vi "HFRR ADV v039.vi"() -> ()   [LabVIEW 2025] (continued)
    n1697 = local read "Calibration Tare Value"() -> (w2060:dbl)
    n1698 = local read "Calibration Tare"() -> (w2058:bool)
    n1699 = Subtract(x=w2056, y=w2060) -> (x-y=→"LVDT STROKE  Calibration":dbl)
    n1700 = case shown="True" w2058 {
      selector: w2058 -> [_ w2066]
      tunnel: w2056 -> [_ w2067]
      frame False {
      }
      frame True {
        n1701 = Not(x=w2066) -> (.not. x?=w2065:bool)
        n1702 = local write "Calibration Tare"(w2065) -> ()
        "Calibration Tare Value" <- w2067
      }
    }
    n1703 = local read "Quit"() -> (w2064:bool)
  }
  n1704 = while {
    stop <- w2090 stop-if-true
    n1705 = local read "Due read"() -> (w2088:string)
    n1706 = call <vilib>:"High Resolution Polling Wait.vi"("seconds to wait"=0.02) -> ()  [unwired: 10 in, 1 out]
    n1707 = local read "Frictioin Force Raw"() -> (w2070:dbl)
    n1708 = Spreadsheet String To Array(delimiter (Tab)=";", format string="", spreadsheet string=w2088, array type (2D Dbl)=string[] []) -> (array=w2085:string[])
    n1709 = Fract/Exp String To Number(string=w2085) -> (number=w2084:dbl[])  [unwired: 3 in, 1 out]
    n1710 = call <vilib>:"Median Filter PtByPt.vi"("rank"=2, "x"=w2070) -> ("Filtered x"=→"Friction":dbl)  [unwired: 2 in, 1 out]
    n1711 = Index Array(array=w2084) -> (element #1=→"Sample Temperature":dbl, element #2=→"Target Sample Temperature":dbl, element #3=→"Current Duty Cycle":dbl, element #4=→"Ambient Temperature":dbl, element #5=→"Dac Status":dbl, element #6=→"Vpp":dbl, element #7=→"Active Error Code":dbl, element #8=→"Kp":dbl, element #9=→"Ki":dbl, element #10=→"Kd":dbl, element #11=→"SampleRaw":dbl, element #12=→"AmbRaw":dbl)  [unwired: 12 in]
    n1712 = local read "Quit"() -> (w2090:bool)
  }
  n1713 = while {
    shift-right: [w2104] -> w41
    shift-left: _ -> [w2096]
    shift-right: [w2091] -> w40
    shift-left: errorcluster {"status"=FALSE, "code"=0, "source"="Init"} ("error out") -> [w2098]
    tunnel: [w2093] -> w44
    tunnel: [w2103] -> _
    i -> [w2103]
    stop <- w2093 stop-if-true
    n1714 = local read "Com Port 2"() -> (w2097:refnum<visa-resource-name>)
    n1715 = local read "Port 2a"() -> (w2099:bool)
    n1716 = Unbundle(w2098) -> ("status"=→"Port 4":bool)  [unwired: 2 out]
    n1717 = call <vilib>:"High Resolution Polling Wait.vi"("seconds to wait"=0.02) -> ()  [unwired: 10 in, 1 out]
    n1718 = local read "Port 4"() -> (w2100:bool)
    n1719 = Not Equal?(x=w2097, y=w2096) -> (x != y?=w2095:bool)
    n1720 = Or(x=w2100, y=w2099) -> (x .or. y?=w2102:bool)
    n1721 = case shown="False" w2102 {
      frame False {
        w2107 = TRUE ("Visible")
        n1722 = property on="Port 2a" class="Bool (strict)"("Visible"=w2107) -> ()  [unwired: 2 in, 2 out]
        n1723 = property on="Port 4" class="Bool (strict)"("Visible"=w2107) -> ()  [unwired: 2 in, 2 out]
      }
      frame True {
        w2108 = TRUE ("Visible")
        n1724 = property on="Port 2a" class="Bool (strict)"("Visible"=w2108) -> ()  [unwired: 2 in, 2 out]
        n1725 = property on="Port 4" class="Bool (strict)"("Visible"=w2108) -> ()  [unwired: 2 in, 2 out]
      }
    }
    n1726 = case shown="True" w2095 {
      tunnel: [w2105 errorcluster {"status"=TRUE, "code"=0, "source"="Init"} ("error out")] -> w2094
      tunnel: w2098 -> [w2105 _]
      frame False {
      }
      frame True {
      }
    }
    n1727 = case shown="No Error" w2094 {
      selector: w2094 -> [w2121 w2152]
      tunnel: [w2114 w2157] -> w2104
      tunnel: [w2122 w2150] -> w2091
      tunnel: w2096 -> [w2123 w2155]
      frame No Error {
        n1728 = property class="Instr" props=["Serial Settings:Number of Bytes at Serial Port"](reference=w2123, error in=w2121) -> (reference out=w2115:refnum<visa-resource-name>, error out=w2120:errorcluster)  [unwired: 1 out]
        n1729 = while {
          tunnel: [w2131] -> w2116
          tunnel: [w2130] -> w2117
          tunnel: w2120 -> [w2129]
          tunnel: w2115 -> [w2128]
          tunnel: [w2127] -> _
          i -> [w2127]
          stop <- TRUE stop-if-true
          n1730 = property class="Instr" props=["Serial Settings:Number of Bytes at Serial Port"](reference=w2128, error in=w2129) -> (reference out=w2133:refnum<visa-resource-name>, error out=w2132:errorcluster)  [unwired: 1 out]
          n1731 = VISA Read(VISA resource name=w2133, byte count=u32 1000, error in (no error)=w2132) -> (VISA resource name out=w2130:refnum<visa-resource-name>, read buffer=→"Due read":string, error out=w2131:errorcluster)  [unwired: 1 out]
        }
        n1732 = local read "Due Write"() -> (w2113:string)
        n1733 = call <vilib>:"Trim Whitespace.vi"("string"=w2113) -> ("trimmed string"=w2112:string)  [unwired: 1 in]
        n1734 = Not Equal?(x=w2112, y="") -> (x != y?=w2118:bool)
        n1735 = VISA Flush I/O Buffer(VISA resource name=w2117) -> (VISA resource name out=w2110:refnum<visa-resource-name>, error out=→"error out 10":errorcluster)  [unwired: 2 in]
        n1736 = case shown="True" w2118 {
          tunnel: w2110 -> [w2135 w2140]
          tunnel: [w2135 w2144] -> w2114
          tunnel: w2116 -> [w2134 w2139]
          tunnel: [w2134 w2142] -> w2122
          tunnel: w2112 -> [_ w2138]
          tunnel: [_ w2141] -> _
          frame False {
            # "DATA  WRITE LOOP"
          }
          frame True {
            n1737 = Concatenate Strings(w2138, "\r\n") -> (w2137:string)
            n1738 = VISA Write(VISA resource name=w2140, write buffer=w2137, error in (no error)=w2139) -> (VISA resource name out=w2144:refnum<visa-resource-name>, return count=w2141:u32, error out=w2143:errorcluster)
            n1739 = flat-sequence {
              tunnel: w2143 -> [w2146]
              tunnel: [w2146] -> w2142
              frame #0 {
                n1740 = local write "Due Write"("" ("Command")) -> ()
                n1741 = Wait (ms)(milliseconds to wait=u32 5) -> ()  [unwired: 1 out]
              }
            }
          }
        }
        "Port 2a" <- TRUE ("Port 2a")
      }
      frame Error {
        w2163 = u16 0 items=["None", "XON/XOFF", "RTS/CTS", "XON/XOFF & RTS/CTS", "DTR/DSR", "XON/XOFF & DTR/DSR"] ("flow control (0:none)  2")
        w2161 = u16 10 items=["1.0"=10, "1.5"=15, "2.0"=20] ("stop bits 2")
        w2159 = u16 0 items=["None", "Odd", "Even", "Mark", "Space"] ("parity 2")
        w2160 = u32 10000  # timeout (10sec)
        n1742 = VISA Clear(VISA resource name=w2155, error in (no error)=w2152) -> (VISA resource name out=w2154:refnum<visa-resource-name>, error out=w2153:errorcluster)
        n1743 = VISA Close(VISA resource name=w2154, error in (no error)=w2153) -> (error out=w2156:errorcluster)
        n1744 = call <vilib>:"Clear Errors.vi"("error in (no error)"=w2156) -> ()  [unwired: 5 in, 2 out]
        n1745 = local write "Port 2a"(FALSE ("Port 2a")) -> ()
        n1746 = local read "Com Port 2"() -> (w2149:refnum<visa-resource-name>)
        "visa due" <- w2149
        n1747 = call-poly "VISA Configure Serial Port"("VISA resource name"=w2149, "timeout (10sec)"=w2160, "baud rate (9600)"=u32 250000 ("baud rate  2"), "data bits (8)"=u16 8 ("data bits  2"), "parity (0:none)"=w2159, "stop bits (10: 1 bit)"=w2161, "flow control (0:none)"=w2163) -> ("VISA resource name out"=w2164:refnum<visa-resource-name>, "error out"=w2165:errorcluster)  [unwired: 7 in]
        n1748 = flat-sequence {
          tunnel: w2164 -> [w2167]
          tunnel: w2165 -> [w2166]
          tunnel: [w2167] -> w2157
          tunnel: [w2166] -> w2150
          frame #0 {
            n1749 = Wait (ms)(milliseconds to wait=u32 50) -> ()  [unwired: 1 out]
          }
        }
        "Residual Due" <- ""
      }
    }
    "error out 9" <- w2091
    n1750 = local read "Quit"() -> (w2093:bool)
    "Error Due" <- w2098
  }
  n1751 = local write "FRICVALZ"(0.0 ("FRICVALZ")) -> ()
  n1752 = property on="RUN" class="Bool (strict)"("Visible"=TRUE) -> ()  [unwired: 2 in, 2 out]
  n1753 = while {
    tunnel: [w2182] -> _
    tunnel: [w2169] -> w54
    i -> [w2182]
    stop <- w2169 stop-if-true
    n1754 = local read "conststatus"() -> (w2173:dbl)
    n1755 = local read "Main Tab"() -> (w2171:T2)
    n1756 = local read "EDIT"() -> (w2188:bool)
    n1757 = local read "Rate"() -> (w2187:dbl)
    n1758 = case shown="True" w2188 {
      tunnel: [FALSE TRUE] -> _
      frame False {
      }
      frame True {
      }
    }
    n1759 = Equal?(x=w2171, y=T29."About" ("Main Tab")) -> (x = y?=w2180:bool)
    n1760 = Equal?(x=w2173, y=0.0) -> (x = y?=w2174:bool)
    n1761 = Divide(x=1.0, y=w2187) -> (x/y=w2183:dbl)
    "Time 2" <- w2183
    n1762 = case shown="True" w2174 {
      frame False {
      }
      frame True {
        # "C:\\WinDucom\\calibrate WO 2391.dcf"
        n1763 = local write "Lan flag"(22) -> ()
        n1764 = local write "conststatus"(10.0 ("rpm value : 2")) -> ()
        n1765 = String To Path(string="C:\\LAB-IQ\\calibrate WO 2465.dcf") -> (path=w2194:path)
        n1766 = Open/Create/Replace File "Open File"(file path (use dialog)=w2194) -> (refnum out=w2192:refnum<file>)  [unwired: 5 in, 2 out]
        n1767 = for {
          N: 23 -> [_]
          tunnel: w2192 -> [w2203]
          i -> [w2197]
          (unwired) TRUE ("line mode (F)")
          n1768 = Read from Text File "Read File"(file (use dialog)=w2203) -> (text=w2202:string)  [unwired: 3 in, 3 out]
          n1769 = Match Pattern(string=w2202, regular expression="]") -> (after substring=w2200:string)  [unwired: 1 in, 3 out]
          n1770 = String Subset(string=w2202, offset (0)=5, length (rest)=10 ("length (rest)")) -> (substring=w2195:string)
          n1771 = Fract/Exp String To Number(string=w2195) -> (number=w2196:dbl)  [unwired: 3 in, 1 out]
          n1772 = Match Pattern(string=w2200, regular expression="-") -> (before substring=w2198:string)  [unwired: 1 in, 3 out]
          n1773 = case shown="10" w2197 {
            tunnel: w2196 -> [_ _ _ _ _ _ _ _ _ _ w2210 _ _ _ _ _ _ _ _ _ _ _ _ _]
            tunnel: w2198 -> [_ _ _ _ w2206 w2207 w2208 _ _ _ _ _ _ _ _ _ _ _ _ _ w2211 w2212 w2213 _]
            frame 0 {
            }
            frame 1 {
            }
            frame 2 {
            }
            frame 3 {
            }
            frame 4 {
              n1774 = local write "Com Port 1"(w2206) -> ()
            }
            frame 5 {
              n1775 = local write "Com Port 2"(w2207) -> ()
              n1776 = local write "visa due"(w2207) -> ()
            }
            frame 6 {
              n1777 = String To Path(string=w2208) -> (path=w2209:path)
              n1778 = local write "File Path"(w2209) -> ()
              "String" <- w2208
            }
            frame 7 {
            }
            frame 8 {
            }
            frame 9 {
            }
            frame 10 {
              n1779 = local write "Language Selection"(w2210) -> ()
            }
            frame 11 {
            }
            frame 12 {
            }
            frame 13 {
            }
            frame 14 {
            }
            frame 15 {
            }
            frame 16 {
            }
            frame 17 {
            }
            frame 18 {
            }
            frame 21 {
            }
            frame 22 {
              n1780 = local write "Com Port 3"(w2211) -> ()
            }
            frame 20 {
              n1781 = local write "Camera Port :"(w2212) -> ()
            }
            frame 19 {
              n1782 = local write "C3 :"(w2213) -> ()
            }
            frame 23, Default {
            }
          }
        }
      }
    }
    n1783 = Select(t=u32 2500 ("milliseconds to wait"), s=w2180, f=u32 500 ("milliseconds to wait")) -> (s? t:f=w2178:u32)
    n1784 = Multiply(x=w2183, y=w2178) -> (x*y=w2185:dbl)
    n1785 = call "Elapsed Time2"("Time Target (s)"=w2185, "Auto Reset"=TRUE) -> ("Time has Elapsed"=w2175:bool)  [unwired: 10 in, 7 out]
    n1786 = case shown="True" w2175 {
      frame False {
      }
      frame True {
        n1787 = stacked-sequence {
          frame #0 {
            # "DATA PROCESSING"
            # "115 mV/N"
            n1788 = local read "Sample Temperature"() -> (w2216:dbl)
            n1789 = local read "RH Numeric:"() -> (→"Humidity ( %RH )":dbl)
            n1790 = local read "FRICVALZ"() -> (w2233:dbl)
            n1791 = local read "Friction"() -> (w2219:dbl)
            n1792 = call <vilib>:"Mean PtByPt.vi"("x"=w2216, "sample length"=100) -> ("mean"=w2215:dbl)  [unwired: 2 in, 1 out]
            "TEMP 2" <- w2215
            "TEMP 3" <- w2215
            n1793 = Subtract(x=w2219, y=w2233) -> (x-y=w2228:dbl)
            "FF 2" <- w2228
            "FF 4" <- w2228
            n1794 = local read "Ambient Temperature"() -> (→"AIR TEMP":dbl)
            n1795 = local read "TEMP"() -> (w2232:dbl)
            n1796 = local write "FF 3"(w2228) -> ()
            n1797 = Compound Arithmetic op=OR("FRICVALZ 4", "FRICVALZ 3", "FRICVALZ 2") -> (w2224:bool)
            n1798 = case shown="True" w2224 {
              tunnel: w2219 -> [_ w2239]
              frame False {
              }
              frame True {
                w2238 = FALSE ("FRICVALZ")
                n1799 = local write "FRICVALZ 3"(w2238) -> ()
                n1800 = local write "FRICVALZ 2"(w2238) -> ()
                n1801 = local write "FRICVALZ 4"(w2238) -> ()
                "FRICVALZ" <- w2239
              }
            }
            n1802 = Not A Number/Path/Refnum?(number/path/refnum=w2232) -> (NaN/Path/Refnum?=w2231:bool)
            n1803 = Not A Number/Path/Refnum?(number/path/refnum=w2228) -> (NaN/Path/Refnum?=w2230:bool)
            n1804 = Divide(x=w2228, y=1.96) -> (x/y=w2225:dbl)
            n1805 = Compound Arithmetic op=OR(w2231, w2230) -> (w2229:bool)
            n1806 = Not A Number/Path/Refnum?(number/path/refnum=w2225) -> (NaN/Path/Refnum?=w2226:bool)
            n1807 = case shown="True" w2229 {
              frame False {
              }
              frame True {
                n1808 = local write "TEMP"(0.0 ("TEMP")) -> ()
                n1809 = local write "FF 2"(0.0 ("FF 2")) -> ()
                n1810 = local write "reinit"(TRUE ("reinit")) -> ()
              }
            }
            n1811 = local write "TEMP"(w2215) -> ()
            n1812 = Select(t=0.0, s=w2226, f=w2225) -> (s? t:f=w2218:dbl)
            "COF 2" <- w2218
            n1813 = local write "COF 3"(w2218) -> ()
          }
        }
      }
    }
    n1814 = Wait (ms)(milliseconds to wait=u32 50) -> ()  [unwired: 1 out]
    n1815 = local read "Quit"() -> (w2169:bool)
    "Rate" <- 2500.0 ("No of Samples")
  }
  n1816 = while {
    tunnel: [w2259] -> _
    tunnel: [w2242] -> w56
    tunnel: w1 -> [_]
    i -> [w2259]
    stop <- w2242 stop-if-true
    # "C:\\LAB-IQ-NXT\\Scar View.exe"
    n1817 = local read "OK Button 16"() -> (w2249:bool)
    n1818 = local read "Main Tab"() -> (w2243:T2)
    n1819 = local read "service 3"() -> (w2244:bool)
    n1820 = local read "OPEN 6"() -> (w2246:bool)
    n1821 = local read "EDIT 2"() -> (w2248:bool)
    n1822 = flat-sequence {
      frame #0 {
        n1823 = stacked-sequence {
          frame #0 {
            n1824 = local read "EDIT"() -> (w2737:bool)
            n1825 = case shown="False" w2737 {
              tunnel: [u8 2 ("Disabled") u8 0 ("Disabled")] -> _
              frame False {
                w2739 = FALSE
                n1826 = local write "Password"("") -> ()
                n1827 = local write "x = y?"(w2739) -> ()
                n1828 = property on="Password" class="Str"("Visible"=w2739) -> ()  [unwired: 2 in, 2 out]
              }
              frame True {
                n1829 = property on="Password" class="Str"("Visible"=TRUE) -> ()  [unwired: 2 in, 2 out]
              }
            }
            "dipl pwd" <- "@143$\n" ("dipl pwd")
          }
          frame #1 {
          }
          frame #2 {
          }
          frame #3 {
          }
          frame #4 {
            n1830 = String To Byte Array(string="Password") -> (unsigned byte array=w2750:u8[])
            n1831 = Search 1D Array(1D array=w2750, element=u8 10) -> (index of element=w2748:i32)  [unwired: 1 in]
            n1832 = Index Array(array=w2750, index=w2748) -> (element=w2749:u8)
            n1833 = Equal?(x=w2749, y=10) -> (x = y?=w2745:bool)
            n1834 = case shown="True" w2745 {
              frame False {
              }
              frame True {
                # "password"
                # "password"
                n1835 = local read "Password"() -> (w2762:string)
                n1836 = String To Byte Array(string=w2762) -> (unsigned byte array=w2765:u8[])
                n1837 = String To Byte Array(string="@143$\n") -> (unsigned byte array=w2752:u8[])
                n1838 = Array Size(array=w2765) -> (size(s)=w2761:i32)
                n1839 = Array Size(array=w2752) -> (size(s)=w2757:i32)
                n1840 = for {
                  N: w2761 -> [_]
                  tunnel: w2765 -> [w2778]
                  tunnel: [w2776] -> w2766 mode=indexing
                  tunnel: w2761 -> [w2773]
                  i -> [w2774]
                  n1841 = Decrement(x=w2773) -> (x-1=w2772:i32)
                  n1842 = Index Array(array=w2778, index=w2774) -> (element=w2777:u8)
                  n1843 = Equal?(x=w2774, y=w2772) -> (x = y?=w2771:bool)
                  n1844 = Number To Decimal String(number=w2777) -> (decimal integer string=w2775:string)  [unwired: 1 in]
                  n1845 = Select(t="", s=w2771, f="\r") -> (s? t:f=w2768:string)
                  n1846 = Concatenate Strings(w2775, w2768) -> (w2776:string)
                }
                n1847 = for {
                  N: w2757 -> [_]
                  tunnel: w2752 -> [w2789]
                  tunnel: [w2787] -> w2755 mode=indexing
                  tunnel: w2757 -> [w2784]
                  i -> [w2785]
                  n1848 = Decrement(x=w2784) -> (x-1=w2783:i32)
                  n1849 = Index Array(array=w2789, index=w2785) -> (element=w2788:u8)
                  n1850 = Equal?(x=w2785, y=w2783) -> (x = y?=w2782:bool)
                  n1851 = Number To Decimal String(number=w2788) -> (decimal integer string=w2786:string)  [unwired: 1 in]
                  n1852 = Select(t="", s=w2782, f="\r") -> (s? t:f=w2779:string)
                  n1853 = Concatenate Strings(w2786, w2779) -> (w2787:string)
                }
                n1854 = local read "file path"() -> (w2751:path)
                n1855 = call <vilib>:"Read Characters From File.vi"("file path (dialog if empty)"=w2751) -> ("character string"=w2764:string)  [unwired: 5 in, 3 out]
                "string" <- w2764
                n1856 = flat-sequence {
                  tunnel: [w2767] -> _
                  frame #0 {
                    w2767 = ""
                    n1857 = local write "Password"(w2767) -> ()
                  }
                }
                n1858 = Concatenate Strings(w2755) -> (w2756:string)
                n1859 = Concatenate Strings(w2764) -> (w2763:string)
                n1860 = Concatenate Strings(w2766) -> (w2759:string)
                n1861 = Equal?(x=w2759, y=w2763) -> (x = y?=w2754:bool)
                n1862 = Equal?(x=w2759, y=w2756) -> (x = y?=w2760:bool)
                n1863 = Or(x=w2754, y=w2760) -> (x .or. y?=→"x = y?":bool)
              }
            }
          }
        }
        n1864 = local read "x = y?"() -> (w2735:bool)
        n1865 = And(x="EDIT", y=w2735) -> (x .and. y?=w2733:bool)
        n1866 = case shown="True" w2733 {
          tunnel: [u8 2 ("Disabled") u8 0 ("Disabled")] -> w2732
          tunnel: [w2939 TRUE ("Visible")] -> w2731
          frame False {
            w2939 = FALSE ("Visible")
            n1867 = local write "EDIT 2"(w2939) -> ()
          }
          frame True {
          }
        }
        n1868 = case shown="True" "SAVE" {
          frame False {
          }
          frame True {
            n1869 = stacked-sequence {
              seq-local: [w2794 _ _] -> [_ w2935 _]
              frame #0 {
                w2790 = 0.0 ("number")
                w2791 = 0.0 ("number")
                (unwired) i16 5 ("precision (6)")
                # "[CH1]    - FF\n[CH2]   - TEMPERATURE\n[CH3]    - Humidity\n[CH4]    - AIR TEMP\n[CH5]\\- Visa Uno\n[CH6] \\- Visa Due\n[CH7]  \\- file path\n[CH8]   - Displacement Gain\n[CHA]   - Stroke Gain\n[CHB]   - Stroke PID Gain\n[CHC]   -Language Selection\n[CHD]   -Power +\n[CHE]   -Power_\n[CHF]   -Heater\n[CHG]   -Humidity Wet\n[CHH]   -Humidity Dry\n[CHI]   -Integral Time"
                n1870 = local read "Language Selection"() -> (w2837:enum16{"English", "Russian"})
                n1871 = Path To String(path="File Path") -> (string=w2853:string)
                n1872 = Number To Fractional String(number=w2790, width (-)=i16 10 ("precision (6)"), precision (6)=i16 5) -> (F-format string=w2844:string)  [unwired: 1 in]
                n1873 = Number To Fractional String(number=w2837, width (-)=i16 10 ("precision (6)"), precision (6)=i16 5) -> (F-format string=w2833:string)  [unwired: 1 in]
                n1874 = Number To Fractional String(number=w2791, width (-)=i16 10 ("precision (6)"), precision (6)=i16 5) -> (F-format string=w2827:string)  [unwired: 1 in]
                n1875 = Number To Fractional String(number=w2791, width (-)=i16 10 ("precision (6)"), precision (6)=i16 5) -> (F-format string=w2824:string)  [unwired: 1 in]
                n1876 = Number To Fractional String(number=w2791, width (-)=i16 10 ("precision (6)"), precision (6)=i16 5) -> (F-format string=w2819:string)  [unwired: 1 in]
                n1877 = Number To Fractional String(number=w2791, width (-)=i16 10 ("precision (6)"), precision (6)=i16 5) -> (F-format string=w2816:string)  [unwired: 1 in]
                n1878 = Number To Fractional String(number=w2791, width (-)=i16 10 ("precision (6)"), precision (6)=i16 5) -> (F-format string=w2811:string)  [unwired: 1 in]
                n1879 = local read "Com Port 1"() -> (w2793:refnum<visa-resource-name>)
                n1880 = local read "Com Port 2"() -> (w2792:refnum<visa-resource-name>)
                n1881 = Concatenate Strings(w2853, "\\" ("string")) -> (w2852:string)
                n1882 = Number To Fractional String(number=w2790, width (-)=i16 10 ("precision (6)"), precision (6)=i16 5) -> (F-format string=w2885:string)  [unwired: 1 in]
                n1883 = Number To Fractional String(number=w2790, width (-)=i16 10 ("precision (6)"), precision (6)=i16 5) -> (F-format string=w2884:string)  [unwired: 1 in]
                n1884 = Number To Fractional String(number=w2790, width (-)=i16 10 ("precision (6)"), precision (6)=i16 5) -> (F-format string=w2878:string)  [unwired: 1 in]
                n1885 = Number To Fractional String(number=w2790, width (-)=i16 10 ("precision (6)"), precision (6)=i16 5) -> (F-format string=w2872:string)  [unwired: 1 in]
                n1886 = Number To Fractional String(number=w2790, width (-)=i16 10 ("precision (6)"), precision (6)=i16 5) -> (F-format string=w2845:string)  [unwired: 1 in]
                n1887 = Concatenate Strings("[CHA]" ("string"), w2844, "- Stroke Gain" ("string"), "\r") -> (w2838:string)
                n1888 = Concatenate Strings("[CHC]" ("string"), w2833, "-Language Selection" ("string"), "\r") -> (w2830:string)
                n1889 = Concatenate Strings("[CHD]" ("string"), w2827, "-Power +" ("string"), "\r") -> (w2809:string)
                n1890 = Concatenate Strings("[CHG]" ("string"), w2816, "-Humidity Wet" ("string"), "\r") -> (w2806:string)
                n1891 = Concatenate Strings("[CHH]" ("string"), w2811, "-Humidity Dry" ("string"), "\r") -> (w2805:string)
                n1892 = Concatenate Strings("[CH1]" ("string"), w2885, " - FF" ("string"), "\r") -> (w2883:string)
                n1893 = Concatenate Strings("[CH2]" ("string"), w2884, " - TEMPERATURE" ("string"), "\r") -> (w2882:string)
                n1894 = Concatenate Strings("[CH3]" ("string"), w2878, " - Humidity" ("string"), "\r") -> (w2875:string)
                n1895 = Concatenate Strings("[CH4]" ("string"), w2872, " - AIR TEMP" ("string"), "\r") -> (w2868:string)
                n1896 = Concatenate Strings("[CH5]" ("string"), w2793, "- Visa Uno" ("string"), "\r") -> (w2861:string)
                n1897 = Concatenate Strings("[CH6]" ("string"), w2792, "- Visa Due" ("string"), "\r") -> (w2856:string)
                n1898 = Concatenate Strings("[CH7]" ("string"), w2852, "- file path" ("string"), "\r") -> (w2855:string)
                n1899 = Concatenate Strings("[CH8]" ("string"), w2845, "- Displacement Gain" ("string"), "\r") -> (w2848:string)
                n1900 = Concatenate Strings("[CHE]" ("string"), w2824, "-Power_" ("string"), "\r") -> (w2808:string)
                n1901 = Concatenate Strings("[CHF]" ("string"), w2819, "-Heater" ("string"), "\r") -> (w2807:string)
                n1902 = Concatenate Strings(w2883, w2882, w2875, w2868, w2861, w2856, w2855, w2848, w2838, w2830, w2809, w2808, w2807, w2806, w2805) -> (w2794:string)
                "gain" <- w2794
              }
              frame #1 {
                w2896 = 0.0 ("number")
                n1903 = local read "Camera Port :"() -> (w2899:string)
                n1904 = local read "C3 :"() -> (w2907:refnum<visa-resource-name>)
                n1905 = local read "Com Port 3"() -> (w2908:refnum<visa-resource-name>)
                n1906 = Concatenate Strings("[CH8]" ("string"), w2899, "- Visa Camera" ("string"), "\r") -> (w2898:string)
                n1907 = Concatenate Strings("[CH7]" ("string"), w2907, "- Visa Humidity" ("string"), "\r") -> (w2903:string)
                n1908 = Number To Fractional String(number=w2896, width (-)=i16 10 ("precision (6)"), precision (6)=i16 5) -> (F-format string=w2923:string)  [unwired: 1 in]
                n1909 = Concatenate Strings("[CHL]" ("string"), w2908, "- Visa humid" ("string"), "\r") -> (w2911:string)
                n1910 = Number To Fractional String(number=w2896, width (-)=i16 10 ("precision (6)"), precision (6)=i16 5) -> (F-format string=w2930:string)  [unwired: 1 in]
                n1911 = Concatenate Strings("[CHK]" ("string"), w2923, "-TEMP INTERCEPT" ("string"), "\r") -> (w2919:string)
                n1912 = Concatenate Strings("[SNO]" ("string"), "" ("string"), "-" ("string"), "\r") -> (w2916:string)
                n1913 = Concatenate Strings("[CHJ]" ("string"), w2930, "-AIR TEMP INTERCEPT" ("string"), "\r") -> (w2920:string)
                n1914 = String To Path(string="C:\\LAB-IQ\\calibrate WO 2465.dcf") -> (path=w2909:path)
                n1915 = Concatenate Strings(w2935, w2920, w2919, w2916, w2911, w2903, w2898) -> (w2934:string)
                n1916 = call <vilib>:"Write Characters To File.vi"("append to file? (new file:F)"=FALSE, "character string"=w2934, "file path (dialog if empty)"=w2909) -> ()  [unwired: 2 in, 1 out]
              }
              frame #2 {
                n1917 = local write "Lan flag"(0.0 ("Lan flag")) -> ()
                n1918 = local write "conststatus"(0.0 ("rpm value : 2")) -> ()
                n1919 = local write "SAVE"(FALSE ("OK Button 14")) -> ()
              }
            }
          }
        }
        n1920 = property on="EDIT 2" class="Bool (strict)"("Visible"=w2731) -> ()  [unwired: 2 in, 2 out]
        n1921 = property on="SAVE" class="Bool (strict)"("Visible"=w2731) -> ()  [unwired: 2 in, 2 out]
        n1922 = property on="visa due" class="CmbBox"("Disabled"=w2732) -> ()  [unwired: 2 in, 2 out]
        n1923 = property on="File Path" class="Path"("Disabled"=w2732) -> ()  [unwired: 2 in, 2 out]
        n1924 = property on="Language Selection" class="Enum (strict)"("Visible"=w2731) -> ()  [unwired: 2 in, 2 out]
        n1925 = property on="SPEED OUT:" class="DigNum (strict)"("Disabled"=w2732) -> ()  [unwired: 2 in, 2 out]
      }
    }
    n1926 = local read "RUN"() -> (w2258:bool)
    n1927 = local read "RUN"() -> (w2256:bool)
    n1928 = case shown="True" "EDIT 3" {
      frame False {
      }
      frame True {
        n1929 = local write "EDIT 3"(FALSE ("EDIT 3")) -> ()
        n1930 = local write "Main Tab"(T2."About" ("Main Tab")) -> ()
      }
    }
    n1931 = case shown="False" w2258 {
      frame False {
        n1932 = local read "stopT"() -> (w2946:bool)
        n1933 = case shown="True" w2946 {
          frame False {
          }
          frame True {
            n1934 = local write "stopT"(FALSE) -> ()
          }
        }
      }
      frame True {
        "stopT" <- TRUE
      }
    }
    n1935 = case shown="False" w2256 {
      frame False {
      }
      frame True {
      }
    }
    n1936 = case shown="True" w2248 {
      frame False {
        n1937 = property on="Password 2" class="Str"("Visible"=FALSE) -> ()  [unwired: 2 in, 2 out]
        n1938 = local write "Password 2"("" ("Password")) -> ()
      }
      frame True {
        n1939 = property on="Password 2" class="Str"("Visible"=TRUE) -> ()  [unwired: 2 in, 2 out]
        n1940 = Equal?(x="Password 2", y="HFRR1234") -> (x = y?=w2271:bool)
        n1941 = case shown="True" w2271 {
          tunnel: "Password 2" -> [w2274 _]
          frame False {
            n1942 = String Length(string=w2274) -> (length=w2275:i32)
            n1943 = Greater Than 0?(x=w2275) -> (x > 0?=w2273:bool)
            n1944 = case shown="False" w2273 {
              frame False {
                n1945 = property on="Password 2" class="Str"("Caption.Text"="Password (Advance Setting)") -> ()  [unwired: 2 in, 2 out]
              }
              frame True {
                n1946 = property on="Password 2" class="Str"("Caption.Text"="Incorrect Password!") -> ()  [unwired: 2 in, 2 out]
              }
            }
          }
          frame True {
            n1947 = local write "EDIT 2"(FALSE ("EDIT 2")) -> ()
            n1948 = local write "Password 2"("" ("Password")) -> ()
            n1949 = local write "Main Tab"(T2."Advance" ("Main Tab")) -> ()
            n1950 = local write "Main Dashboard Buttons"(T1."Advance" ("Main Dashboard Buttons")) -> ()
          }
        }
      }
    }
    n1951 = case shown="True" "Prog Uno" {
      frame False {
      }
      frame True {
        n1952 = stacked-sequence {
          frame #0 {
            n1953 = Delete(path (use dialog)=path "C:/LAB-IQ-NXT/UNOCOMPILE.bat" ("working directory")) -> ()  [unwired: 4 in, 3 out]
          }
          frame #1 {
            n1954 = local read "Com Port 1"() -> (w2713:refnum<visa-resource-name>)
            n1955 = Concatenate Strings("cmd.exe /c \"mode " ("command line"), w2713, ":1200,n,8,1\"\n" ("command line")) -> (w2718:string)
            n1956 = Concatenate Strings(w2718, "CD\\\nCD WinDucom\navrdude -C avrdude.conf -v -patmega328p -carduino -P" ("command line"), w2713, " -b115200 -D -Uflash:w:UNO_V20.hex:i\n" ("command line"), "\r") -> (w2720:string)
            "STR" <- w2720
            n1957 = call <vilib>:"Write Characters To File.vi"("append to file? (new file:F)"=FALSE, "character string"=w2720, "file path (dialog if empty)"=path "C:/LAB-IQ/UNOCOMPILE.bat" ("working directory")) -> ()  [unwired: 2 in, 1 out]
          }
          frame #2 {
            n1958 = disable-structure shown="Disabled" {
              frame Disabled {
                w2724 = "cmd.exe  /c \"C:\\LAB-IQ-NXT\\UNOCOMPILE.bat\"" ("string")
                n1959 = local write "Prog Uno"(FALSE ("run minimized? (F)")) -> ()
                n1960 = call <vilib>:"System Exec.vi"("expected output size  (4096)"=u32 65535, "run minimized? (F)"=FALSE, "wait until completion? (T)"=TRUE ("run minimized? (F)"), "working directory"=path "C:/LAB-IQ-NXT", "standard input"=w2724, "command line"=w2724) -> ("error out"=w2723:errorcluster, "standard output"=→"String 42":string)  [unwired: 2 in, 2 out]
                "error out 3" <- w2723
                n1961 = flat-sequence {
                  tunnel: w2723 -> [_]
                  frame #0 {
                  }
                }
              }
              frame Enabled {
              }
            }
          }
        }
      }
    }
    n1962 = case shown="\"ISO 12156\"" "TEST STANDARD" {
      frame "ASTM D6079", Default {
        w2693 = 50.0 ("Hz")
        w2694 = 53.0 ("Set Rh")
        w2696 = 1.0 ("Set Strk")
        w2695 = 60.0 ("Set Temp")
        # "astm hide"
        n1963 = local write "NORMAL LOAD"(200.0 ("NORMAL LOAD")) -> ()
        n1964 = local write "Set Strk"(w2696) -> ()
        n1965 = local write "Set Hz"(w2693) -> ()
        n1966 = local write "Set Temp"(w2695) -> ()
        n1967 = local write "Set Rh"(w2694) -> ()
        n1968 = local write "test time"(75.0 ("test time")) -> ()
        n1969 = local write "Set Stroke:"(w2696) -> ()
        n1970 = local write "Set Humidity:"(w2694) -> ()
        n1971 = local write "Set Frequency:"(w2693) -> ()
        n1972 = local write "Set Temperature:"(w2695) -> ()
        "Test Standard" <- "ASTM D6079" ("Test Standard 2")
      }
      frame "ISO 12156" {
        n1973 = local write "Set Strk"(1.0 ("Set Strk")) -> ()
        n1974 = local write "NORMAL LOAD"(200.0 ("NORMAL LOAD")) -> ()
        n1975 = local write "Set Temp"(60.0 ("Set Temp")) -> ()
        n1976 = local write "test time"(75.0 ("test time")) -> ()
        n1977 = local write "Set Hz"(50.0 ("Hz")) -> ()
        n1978 = local write "Set Rh"(53.0 ("Set Rh")) -> ()
      }
      frame "CEC F-096-A-06" {
        n1979 = local write "Set Strk"(1.0 ("Set Strk")) -> ()
        n1980 = local write "NORMAL LOAD"(200.0 ("NORMAL LOAD")) -> ()
        n1981 = local write "Set Temp"(60.0 ("Set Temp")) -> ()
        n1982 = local write "test time"(75.0 ("test time")) -> ()
        n1983 = local write "Set Hz"(50.0 ("Hz")) -> ()
        n1984 = local write "Set Rh"(53.0 ("Set Rh")) -> ()
      }
      frame "Custom" {
      }
    }
    n1985 = Or(x=w2246, y=w2244) -> (x .or. y?=w2245:bool)
    n1986 = case shown="\"About\"" w2243 {
      tunnel: [T29."Acquire" ("Main Tab") T29."Compare Files" ("Main Tab") T29."About" ("Main Tab")] -> w2254
      frame "Acquire", Default {
      }
      frame "Compare Files" {
      }
      frame "About" {
      }
    }
    n1987 = Or(x=w2249, y="OPEN") -> (x .or. y?=w2250:bool)
    n1988 = case shown="True" w2250 {
      tunnel: w2249 -> [_ w2282]
      frame False {
      }
      frame True {
        n1989 = stacked-sequence {
          tunnel: w2282 -> [_ w2349 _ _]
          frame #0 {
            w2298 = "  " ("String 6")
            n1990 = local write "OPEN"(FALSE ("open")) -> ()
            n1991 = local read "string1 2"() -> (w2286:string)
            n1992 = local read "string1 3"() -> (w2285:string)
            n1993 = local read "string1 4"() -> (w2284:string)
            n1994 = property on="OPEN" class="Bool (strict)"("Visible"=FALSE) -> ()  [unwired: 2 in, 2 out]
            n1995 = local write "String 6"(w2298) -> ()
            n1996 = local write "String 7"(w2298) -> ()
            n1997 = local write "String 8"(w2298) -> ()
            n1998 = local write "String 12"(w2298) -> ()
            n1999 = local read "OK Button 16"() -> (w2283:bool)
            n2000 = String To Path(string=w2286) -> (path=w2294:path)
            n2001 = String To Path(string=w2285) -> (path=w2293:path)
            n2002 = String To Path(string=w2284) -> (path=w2292:path)
            n2003 = case shown="True" w2283 {
              tunnel: [w2299 w2300] -> w2287
              frame False {
                n2004 = local read "string1"() -> (w2299:string)
              }
              frame True {
                n2005 = local read "String Indicator 4"() -> (w2300:string)
              }
            }
            n2006 = Open/Create/Replace File "Open File"(file path (use dialog)=w2294) -> (refnum out=w2290:refnum<file>)  [unwired: 5 in, 2 out]
            n2007 = Open/Create/Replace File "Open File"(file path (use dialog)=w2293) -> (refnum out=w2289:refnum<file>)  [unwired: 5 in, 2 out]
            n2008 = Open/Create/Replace File "Open File"(file path (use dialog)=w2292) -> (refnum out=w2288:refnum<file>)  [unwired: 5 in, 2 out]
            n2009 = while {
              tunnel: w2290 -> [w2312]
              i -> [w2308]
              stop <- w2307 continue-if-true
              (unwired) TRUE ("line mode (F)")
              n2010 = Read from Text File "Read File"(file (use dialog)=w2312) -> (text=w2309:string)  [unwired: 3 in, 3 out]
              n2011 = local write "Numeric 11"(w2308) -> ()
              n2012 = String Length(string=w2309) -> (length=w2311:i32)
              n2013 = Greater?(x=w2311, y=1) -> (0:w2307:bool)
            }
            n2014 = while {
              tunnel: w2289 -> [w2318]
              i -> [w2314]
              stop <- w2313 continue-if-true
              (unwired) TRUE ("line mode (F)")
              n2015 = Read from Text File "Read File"(file (use dialog)=w2318) -> (text=w2315:string)  [unwired: 3 in, 3 out]
              n2016 = local write "Numeric 12"(w2314) -> ()
              n2017 = String Length(string=w2315) -> (length=w2317:i32)
              n2018 = Greater?(x=w2317, y=1) -> (0:w2313:bool)
            }
            n2019 = while {
              tunnel: w2288 -> [w2324]
              i -> [w2320]
              stop <- w2319 continue-if-true
              (unwired) TRUE ("line mode (F)")
              n2020 = Read from Text File "Read File"(file (use dialog)=w2324) -> (text=w2321:string)  [unwired: 3 in, 3 out]
              n2021 = local write "Numeric 13"(w2320) -> ()
              n2022 = String Length(string=w2321) -> (length=w2323:i32)
              n2023 = Greater?(x=w2323, y=1) -> (0:w2319:bool)
            }
            n2024 = String To Path(string=w2287) -> (path=w2295:path)
            n2025 = Open/Create/Replace File "Open File"(file path (use dialog)=w2295) -> (refnum out=w2291:refnum<file>)  [unwired: 5 in, 2 out]
            n2026 = while {
              tunnel: w2291 -> [w2306]
              i -> [w2302]
              stop <- w2301 continue-if-true
              (unwired) TRUE ("line mode (F)")
              n2027 = Read from Text File "Read File"(file (use dialog)=w2306) -> (text=w2303:string)  [unwired: 3 in, 3 out]
              n2028 = local write "Numeric 8"(w2302) -> ()
              n2029 = String Length(string=w2303) -> (length=w2305:i32)
              n2030 = Greater?(x=w2305, y=1) -> (0:w2301:bool)
            }
          }
          frame #1 {
            w2476 = FALSE ("ACTUAL   MERGE")
            # "Sample Temp"
            # "ECR"
            # "COF"
            # "Time\nCOF\nFF\nTemp"
            n2031 = case shown="True" w2349 {
              tunnel: [w2496 w2497] -> w2350
              frame False {
                n2032 = local read "string1"() -> (w2496:string)
              }
              frame True {
                n2033 = local read "String Indicator 4"() -> (w2497:string)
              }
            }
            n2034 = local read "string1 3"() -> (w2394:string)
            n2035 = String To Path(string=w2350) -> (path=w2481:path)
            n2036 = String To Path(string=w2394) -> (path=w2492:path)
            n2037 = local read "Numeric 12"() -> (w2478:i32)
            n2038 = local read "Numeric 8"() -> (w2480:i32)
            n2039 = local read "string1 2"() -> (w2395:string)
            n2040 = local read "string1 4"() -> (w2393:string)
            n2041 = Open/Create/Replace File "Open File"(file path (use dialog)=w2481) -> (refnum out=w2495:refnum<file>, error out=w2494:errorcluster)  [unwired: 5 in, 1 out]
            n2042 = Open/Create/Replace File "Open File"(file path (use dialog)=w2492) -> (refnum out=w2488:refnum<file>, error out=w2489:errorcluster)  [unwired: 5 in, 1 out]
            n2043 = for {
              N: w2480 -> [_]
              tunnel: w2495 -> [w2643]
              tunnel: w2494 -> [w2642]
              tunnel: [w2632] -> w2407 mode=indexing
              tunnel: [w2630] -> w2464 mode=indexing
              tunnel: [w2631] -> w2459 mode=indexing
              tunnel: w2476 -> [_]
              tunnel: [w2624] -> w2461 mode=indexing
              tunnel: [w2620] -> w2430 mode=indexing
              tunnel: [w2616] -> w2405 mode=indexing
              tunnel: [w2612] -> w2386 mode=indexing
              tunnel: [w2607] -> w2346 mode=indexing
              (unwired) TRUE ("line mode (F)")
              # "freq"
              # "Stroke"
              # "Time"
              # "CoF"
              # "Humidity"
              # "Temp"
              # "Air Temp"
              # "ECR"
              n2044 = Read from Text File "Read File"(file (use dialog)=w2643, error in=w2642) -> (text=w2608:string)  [unwired: 2 in, 3 out]
              n2045 = local write "String 6"(w2608) -> ()
              n2046 = String Subset(string=w2608, offset (0)=0, length (rest)=14 ("length (rest)")) -> (substring=w2636:string)
              n2047 = String Subset(string=w2608, offset (0)=35, length (rest)=9 ("length (rest)")) -> (substring=w2633:string)
              n2048 = String Subset(string=w2608, offset (0)=15, length (rest)=9 ("length (rest)")) -> (substring=w2639:string)
              n2049 = Fract/Exp String To Number(string=w2636) -> (number=w2632:dbl)  [unwired: 3 in, 1 out]
              n2050 = Fract/Exp String To Number(string=w2633) -> (number=w2631:dbl)  [unwired: 3 in, 1 out]
              n2051 = Fract/Exp String To Number(string=w2639) -> (number=w2630:dbl)  [unwired: 3 in, 1 out]
              n2052 = String Subset(string=w2608, offset (0)=85, length (rest)=9 ("length (rest)")) -> (substring=w2609:string)
              n2053 = String Subset(string=w2608, offset (0)=25, length (rest)=9 ("length (rest)")) -> (substring=w2615:string)
              n2054 = String Subset(string=w2608, offset (0)=55, length (rest)=9 ("length (rest)")) -> (substring=w2617:string)
              n2055 = String Subset(string=w2608, offset (0)=45, length (rest)=9 ("length (rest)")) -> (substring=w2623:string)
              n2056 = String Subset(string=w2608, offset (0)=65, length (rest)=9 ("length (rest)")) -> (substring=w2629:string)
              n2057 = Fract/Exp String To Number(string=w2615) -> (number=w2612:dbl)  [unwired: 3 in, 1 out]
              n2058 = Fract/Exp String To Number(string=w2609) -> (number=w2607:dbl)  [unwired: 3 in, 1 out]
              n2059 = Fract/Exp String To Number(string=w2617) -> (number=w2616:dbl)  [unwired: 3 in, 1 out]
              n2060 = Fract/Exp String To Number(string=w2623) -> (number=w2620:dbl)  [unwired: 3 in, 1 out]
              n2061 = Fract/Exp String To Number(string=w2629) -> (number=w2626:dbl)  [unwired: 3 in, 1 out]
              n2062 = Add(x=w2626, y=0.0) -> (x+y=w2624:dbl)
            }
            n2063 = for {
              N: w2478 -> [_]
              tunnel: w2489 -> [w2569]
              tunnel: w2488 -> [w2568]
              tunnel: [w2558] -> w2447 mode=indexing
              tunnel: [w2556] -> w2445 mode=indexing
              tunnel: [w2557] -> w2441 mode=indexing
              tunnel: w2476 -> [_]
              tunnel: [w2550] -> w2443 mode=indexing
              tunnel: [w2546] -> w2425 mode=indexing
              tunnel: [w2542] -> w2401 mode=indexing
              tunnel: [w2539] -> w2382 mode=indexing
              tunnel: [w2535] -> w2341 mode=indexing
              (unwired) 9 ("length (rest)")
              (unwired) 9 ("length (rest)")
              (unwired) TRUE ("line mode (F)")
              n2064 = Read from Text File "Read File"(file (use dialog)=w2568, error in=w2569) -> (text=w2536:string)  [unwired: 2 in, 3 out]
              n2065 = local write "String 8"(w2536) -> ()
              n2066 = String Subset(string=w2536, offset (0)=85) -> (substring=w2538:string)  [unwired: 1 in]
              n2067 = String Subset(string=w2536, offset (0)=35, length (rest)=9 ("length (rest)")) -> (substring=w2559:string)
              n2068 = String Subset(string=w2536, offset (0)=55, length (rest)=9 ("length (rest)")) -> (substring=w2544:string)
              n2069 = String Subset(string=w2536, offset (0)=25) -> (substring=w2540:string)  [unwired: 1 in]
              n2070 = String Subset(string=w2536, offset (0)=15, length (rest)=9 ("length (rest)")) -> (substring=w2565:string)
              n2071 = String Subset(string=w2536, offset (0)=0, length (rest)=14 ("length (rest)")) -> (substring=w2562:string)
              n2072 = String Subset(string=w2536, offset (0)=45, length (rest)=9 ("length (rest)")) -> (substring=w2549:string)
              n2073 = String Subset(string=w2536, offset (0)=65, length (rest)=9 ("length (rest)")) -> (substring=w2555:string)
              n2074 = Fract/Exp String To Number(string=w2538) -> (number=w2535:dbl)  [unwired: 3 in, 1 out]
              n2075 = Fract/Exp String To Number(string=w2559) -> (number=w2557:dbl)  [unwired: 3 in, 1 out]
              n2076 = Fract/Exp String To Number(string=w2544) -> (number=w2542:dbl)  [unwired: 3 in, 1 out]
              n2077 = Fract/Exp String To Number(string=w2540) -> (number=w2539:dbl)  [unwired: 3 in, 1 out]
              n2078 = Fract/Exp String To Number(string=w2565) -> (number=w2556:dbl)  [unwired: 3 in, 1 out]
              n2079 = Fract/Exp String To Number(string=w2562) -> (number=w2558:dbl)  [unwired: 3 in, 1 out]
              n2080 = Fract/Exp String To Number(string=w2549) -> (number=w2546:dbl)  [unwired: 3 in, 1 out]
              n2081 = Fract/Exp String To Number(string=w2555) -> (number=w2552:dbl)  [unwired: 3 in, 1 out]
              n2082 = Add(x=w2552, y=0.0) -> (x+y=w2550:dbl)
            }
            n2083 = String To Path(string=w2395) -> (path=w2493:path)
            n2084 = String To Path(string=w2393) -> (path=w2487:path)
            n2085 = local read "Numeric 11"() -> (w2477:i32)
            n2086 = local read "Numeric 13"() -> (w2479:i32)
            n2087 = Open/Create/Replace File "Open File"(file path (use dialog)=w2493) -> (refnum out=w2491:refnum<file>, error out=w2490:errorcluster)  [unwired: 5 in, 1 out]
            n2088 = Open/Create/Replace File "Open File"(file path (use dialog)=w2487) -> (refnum out=w2486:refnum<file>, error out=w2485:errorcluster)  [unwired: 5 in, 1 out]
            n2089 = for {
              N: w2477 -> [_]
              tunnel: w2491 -> [w2606]
              tunnel: w2490 -> [w2605]
              tunnel: [w2595] -> w2457 mode=indexing
              tunnel: [w2593] -> w2455 mode=indexing
              tunnel: [w2594] -> w2450 mode=indexing
              tunnel: w2476 -> [_]
              tunnel: [w2587] -> w2452 mode=indexing
              tunnel: [w2583] -> w2428 mode=indexing
              tunnel: [w2579] -> w2403 mode=indexing
              tunnel: [w2575] -> w2384 mode=indexing
              tunnel: [w2570] -> w2342 mode=indexing
              (unwired) TRUE ("line mode (F)")
              n2090 = Read from Text File "Read File"(file (use dialog)=w2606, error in=w2605) -> (text=w2571:string)  [unwired: 2 in, 3 out]
              n2091 = local write "String 7"(w2571) -> ()
              n2092 = String Subset(string=w2571, offset (0)=85, length (rest)=9 ("length (rest)")) -> (substring=w2574:string)
              n2093 = String Subset(string=w2571, offset (0)=35, length (rest)=9 ("length (rest)")) -> (substring=w2596:string)
              n2094 = String Subset(string=w2571, offset (0)=55, length (rest)=9 ("length (rest)")) -> (substring=w2582:string)
              n2095 = String Subset(string=w2571, offset (0)=25, length (rest)=9 ("length (rest)")) -> (substring=w2576:string)
              n2096 = String Subset(string=w2571, offset (0)=45, length (rest)=9 ("length (rest)")) -> (substring=w2584:string)
              n2097 = String Subset(string=w2571, offset (0)=0, length (rest)=14 ("length (rest)")) -> (substring=w2599:string)
              n2098 = String Subset(string=w2571, offset (0)=15, length (rest)=9 ("length (rest)")) -> (substring=w2602:string)
              n2099 = String Subset(string=w2571, offset (0)=65, length (rest)=9 ("length (rest)")) -> (substring=w2588:string)
              n2100 = Fract/Exp String To Number(string=w2574) -> (number=w2570:dbl)  [unwired: 3 in, 1 out]
              n2101 = Fract/Exp String To Number(string=w2596) -> (number=w2594:dbl)  [unwired: 3 in, 1 out]
              n2102 = Fract/Exp String To Number(string=w2582) -> (number=w2579:dbl)  [unwired: 3 in, 1 out]
              n2103 = Fract/Exp String To Number(string=w2576) -> (number=w2575:dbl)  [unwired: 3 in, 1 out]
              n2104 = Fract/Exp String To Number(string=w2584) -> (number=w2583:dbl)  [unwired: 3 in, 1 out]
              n2105 = Fract/Exp String To Number(string=w2599) -> (number=w2595:dbl)  [unwired: 3 in, 1 out]
              n2106 = Fract/Exp String To Number(string=w2602) -> (number=w2593:dbl)  [unwired: 3 in, 1 out]
              n2107 = Fract/Exp String To Number(string=w2588) -> (number=w2591:dbl)  [unwired: 3 in, 1 out]
              n2108 = Add(x=w2591, y=0.0) -> (x+y=w2587:dbl)
            }
            n2109 = for {
              N: w2479 -> [_]
              tunnel: w2486 -> [w2534]
              tunnel: w2485 -> [w2533]
              tunnel: [w2523] -> w2439 mode=indexing
              tunnel: [w2522] -> w2432 mode=indexing
              tunnel: w2476 -> [_]
              tunnel: [w2511] -> w2437 mode=indexing
              tunnel: [w2516] -> w2434 mode=indexing
              tunnel: [w2512] -> w2424 mode=indexing
              tunnel: [w2507] -> w2399 mode=indexing
              tunnel: [w2503] -> w2380 mode=indexing
              tunnel: [w2498] -> w2340 mode=indexing
              (unwired) 1.0 ("x")
              (unwired) TRUE ("line mode (F)")
              n2110 = Read from Text File "Read File"(file (use dialog)=w2534, error in=w2533) -> (text=w2499:string)  [unwired: 2 in, 3 out]
              n2111 = local write "String 12"(w2499) -> ()
              n2112 = String Subset(string=w2499, offset (0)=85, length (rest)=9 ("length (rest)")) -> (substring=w2501:string)
              n2113 = String Subset(string=w2499, offset (0)=35, length (rest)=9 ("length (rest)")) -> (substring=w2524:string)
              n2114 = String Subset(string=w2499, offset (0)=55, length (rest)=9 ("length (rest)")) -> (substring=w2509:string)
              n2115 = String Subset(string=w2499, offset (0)=25, length (rest)=9 ("length (rest)")) -> (substring=w2505:string)
              n2116 = String Subset(string=w2499, offset (0)=45, length (rest)=9 ("length (rest)")) -> (substring=w2514:string)
              n2117 = String Subset(string=w2499, offset (0)=15, length (rest)=9 ("length (rest)")) -> (substring=w2530:string)
              n2118 = String Subset(string=w2499, offset (0)=0, length (rest)=14 ("length (rest)")) -> (substring=w2527:string)
              n2119 = String Subset(string=w2499, offset (0)=65, length (rest)=9 ("length (rest)")) -> (substring=w2517:string)
              n2120 = Fract/Exp String To Number(string=w2501) -> (number=w2498:dbl)  [unwired: 3 in, 1 out]
              n2121 = Fract/Exp String To Number(string=w2524) -> (number=w2522:dbl)  [unwired: 3 in, 1 out]
              n2122 = Fract/Exp String To Number(string=w2509) -> (number=w2507:dbl)  [unwired: 3 in, 1 out]
              n2123 = Fract/Exp String To Number(string=w2505) -> (number=w2503:dbl)  [unwired: 3 in, 1 out]
              n2124 = Fract/Exp String To Number(string=w2514) -> (number=w2512:dbl)  [unwired: 3 in, 1 out]
              n2125 = Fract/Exp String To Number(string=w2530) -> (number=w2511:dbl)  [unwired: 3 in, 1 out]
              n2126 = Fract/Exp String To Number(string=w2527) -> (number=w2523:dbl)  [unwired: 3 in, 1 out]
              n2127 = Fract/Exp String To Number(string=w2517) -> (number=w2520:dbl)  [unwired: 3 in, 1 out]
              n2128 = Add(x=w2520, y=0.0) -> (x+y=w2516:dbl)
            }
            n2129 = Delete From Array(array=w2382, index=0) -> (array with subset deleted=w2355:dbl[])  [unwired: 1 in, 1 out]
            n2130 = Delete From Array(array=w2445, index=0) -> (array with subset deleted=w2418:dbl[])  [unwired: 1 in, 1 out]
            n2131 = Delete From Array(array=w2425, index=0) -> (array with subset deleted=w2413:dbl[])  [unwired: 1 in, 1 out]
            n2132 = Delete From Array(array=w2443, index=0) -> (array with subset deleted=w2444:dbl[])  [unwired: 1 in, 1 out]
            n2133 = call-poly <vilib>:"Mean.vi"("X"=w2355) -> ("mean"=→"КОФ2 4":dbl)  [unwired: 1 out]
            n2134 = call-poly <vilib>:"Mean.vi"("X"=w2418) -> ("mean"=→"КОФ3":dbl)  [unwired: 1 out]
            n2135 = call-poly <vilib>:"Mean.vi"("X"=w2413) -> ("mean"=→"CP3":dbl)  [unwired: 1 out]
            n2136 = Delete From Array(array=w2407, index=0) -> (array with subset deleted=w2334:dbl[])  [unwired: 1 in, 1 out]
            n2137 = Delete From Array(array=w2346, index=0) -> (array with subset deleted=w2333:dbl[])  [unwired: 1 in, 1 out]
            n2138 = Delete From Array(array=w2386, index=0) -> (array with subset deleted=w2357:dbl[])  [unwired: 1 in, 1 out]
            n2139 = Delete From Array(array=w2464, index=0) -> (array with subset deleted=w2419:dbl[])  [unwired: 1 in, 1 out]
            n2140 = Delete From Array(array=w2430, index=0) -> (array with subset deleted=w2415:dbl[])  [unwired: 1 in, 1 out]
            "array w/ subset deleted" <- w2415
            n2141 = Delete From Array(array=w2461, index=0) -> (array with subset deleted=w2462:dbl[])  [unwired: 1 in, 1 out]
            n2142 = call-poly <vilib>:"Mean.vi"("X"=w2357) -> ("mean"=→"КОФ2 2":dbl)  [unwired: 1 out]
            n2143 = call-poly <vilib>:"Mean.vi"("X"=w2419) -> ("mean"=→"КОФ1":dbl)  [unwired: 1 out]
            n2144 = Bundle "Bundle"(w2334, w2333) -> (w2339:cluster{dbl[], dbl[]})  [unwired: 1 in]
            n2145 = Bundle "Bundle"(w2334, w2462) -> (w2326:cluster{dbl[], dbl[]})  [unwired: 1 in]
            n2146 = Delete From Array(array=w2341, index=0) -> (array with subset deleted=w2329:dbl[])  [unwired: 1 in, 1 out]
            n2147 = Delete From Array(array=w2342, index=0) -> (array with subset deleted=w2331:dbl[])  [unwired: 1 in, 1 out]
            n2148 = Delete From Array(array=w2452, index=0) -> (array with subset deleted=w2453:dbl[])  [unwired: 1 in, 1 out]
            n2149 = Delete From Array(array=w2340, index=0) -> (array with subset deleted=w2327:dbl[])  [unwired: 1 in, 1 out]
            n2150 = Delete From Array(array=w2434, index=0) -> (array with subset deleted=w2435:dbl[])  [unwired: 1 in, 1 out]
            n2151 = Delete From Array(array=w2459, index=0) -> (array with subset deleted=w2365:dbl[])  [unwired: 1 in, 1 out]
            n2152 = Delete From Array(array=w2405, index=0) -> (array with subset deleted=w2361:dbl[])  [unwired: 1 in, 1 out]
            n2153 = Delete From Array(array=w2441, index=0) -> (array with subset deleted=w2363:dbl[])  [unwired: 1 in, 1 out]
            n2154 = Delete From Array(array=w2401, index=0) -> (array with subset deleted=w2359:dbl[])  [unwired: 1 in, 1 out]
            n2155 = Delete From Array(array=w2450, index=0) -> (array with subset deleted=w2364:dbl[])  [unwired: 1 in, 1 out]
            n2156 = Delete From Array(array=w2403, index=0) -> (array with subset deleted=w2360:dbl[])  [unwired: 1 in, 1 out]
            n2157 = Delete From Array(array=w2384, index=0) -> (array with subset deleted=w2356:dbl[])  [unwired: 1 in, 1 out]
            n2158 = Delete From Array(array=w2428, index=0) -> (array with subset deleted=w2414:dbl[])  [unwired: 1 in, 1 out]
            n2159 = Delete From Array(array=w2455, index=0) -> (array with subset deleted=w2416:dbl[])  [unwired: 1 in, 1 out]
            n2160 = Delete From Array(array=w2432, index=0) -> (array with subset deleted=w2362:dbl[])  [unwired: 1 in, 1 out]
            n2161 = Delete From Array(array=w2399, index=0) -> (array with subset deleted=w2358:dbl[])  [unwired: 1 in, 1 out]
            n2162 = Delete From Array(array=w2380, index=0) -> (array with subset deleted=w2354:dbl[])  [unwired: 1 in, 1 out]
            n2163 = Delete From Array(array=w2424, index=0) -> (array with subset deleted=w2412:dbl[])  [unwired: 1 in, 1 out]
            n2164 = Delete From Array(array=w2437, index=0) -> (array with subset deleted=w2417:dbl[])  [unwired: 1 in, 1 out]
            n2165 = Delete From Array(array=w2447, index=0) -> (array with subset deleted=w2330:dbl[])  [unwired: 1 in, 1 out]
            n2166 = Delete From Array(array=w2457, index=0) -> (array with subset deleted=w2332:dbl[])  [unwired: 1 in, 1 out]
            n2167 = Delete From Array(array=w2439, index=0) -> (array with subset deleted=w2328:dbl[])  [unwired: 1 in, 1 out]